vi "run_pharmaBotExp_v1.000.vi"(0 "data in":T12={"daq_ao 1"="Dev1/ao0", "daq_ai 1"="Dev1/ai0", "experiment day folder"=path "C:/multiBot/data/debug/testing", "Multiclamp init error"=0, "Multiclamp Handle Out"=10225184, "sampling rate (Hz)"=20000, "trial name"="t1"}, 1 "auto run?":bool, 3 "which manipulator":T13(ring), 4 "HEK/slice options":enum16{"slice", "HEK"}(ring), 5 "error in":errorcluster, 6 "Validate after Experiment":bool, 7 "common cluster":T9, 11 "individual controls in":T8, 13 "images":T3={"slice image"="remote image 00000000137F745C", "pipette template"="remote image 00000000137F7D5C", "found pipette"=refnum, "pipette mask for cell tracker"=refnum, "cell images ref"=refnum}) -> (10 "Cell Looks Good?":bool=TRUE, 12 "ValidationOutputCluster":T5(array[cluster]), 14 "ValidationResults":waveform(dbl)[][](array[waveform]), 15 "ValidationPos1":T6(array[ring]), 16 "Exp. Terminated":bool, 17 "ValidationPos2":T6(array[ring]), 18 "ValidationWaveform":waveform(dbl)[](array[waveform]), 19 "error out":errorcluster)   [LabVIEW 2019] (continued)
                  }
                  frame True {
                    n489 = local write "Current Position"(w583) -> ()
                  }
                }
              }
              frame #3 {
                n490 = Unbundle By Name(w601) -> ("JumperPositions.JumperPos A"=w600:refnum<vi>)
                n491 = property class="Arr (strict)"(reference=w600) -> ("Value"=w584:dbl[], "Caption.Text"=w589:string)  [unwired: 1 in, 2 out]
                n492 = Index Array(array=w587) -> (element #1=w598:i32, element #2=w596:i32, element #3=w595:i32)  [unwired: 3 in]
                n493 = Divide(x=w584, y=10) -> (x/y=w585:dbl[])
                n494 = To Long Integer(number=w585) -> (32bit integer=w586:i32[])
                n495 = Index Array(array=w586) -> (element #1=w599:i32, element #2=w597:i32, element #3=w594:i32)  [unwired: 3 in]
                n496 = Equal?(x=w599, y=w598) -> (x = y?=w593:bool)
                n497 = Equal?(x=w597, y=w596) -> (x = y?=w592:bool)
                n498 = Equal?(x=w594, y=w595) -> (x = y?=w591:bool)
                n499 = Compound Arithmetic op=AND(w593, w592, w591) -> (w590:bool)
                n500 = case shown="True" w590 {
                  tunnel: w589 -> [_ w602]
                  frame False {
                  }
                  frame True {
                    n501 = local write "Current Position"(w602) -> ()
                  }
                }
              }
              frame #4 {
                n502 = Unbundle By Name(w620) -> ("JumperPositions.JumperPos B"=w619:refnum<vi>)
                n503 = property class="Arr (strict)"(reference=w619) -> ("Value"=w605:dbl[], "Caption.Text"=w608:string)  [unwired: 1 in, 2 out]
                n504 = Index Array(array=w603) -> (element #1=w617:i32, element #2=w615:i32, element #3=w614:i32)  [unwired: 3 in]
                n505 = Divide(x=w605, y=10) -> (x/y=w606:dbl[])
                n506 = To Long Integer(number=w606) -> (32bit integer=w604:i32[])
                n507 = Index Array(array=w604) -> (element #1=w618:i32, element #2=w616:i32, element #3=w613:i32)  [unwired: 3 in]
                n508 = Equal?(x=w618, y=w617) -> (x = y?=w612:bool)
                n509 = Equal?(x=w616, y=w615) -> (x = y?=w611:bool)
                n510 = Equal?(x=w613, y=w614) -> (x = y?=w610:bool)
                n511 = Compound Arithmetic op=AND(w612, w611, w610) -> (w609:bool)
                n512 = case shown="True" w609 {
                  tunnel: w608 -> [_ w621]
                  frame False {
                  }
                  frame True {
                    n513 = local write "Current Position"(w621) -> ()
                  }
                }
              }
              frame #5 {
                n514 = Unbundle By Name(w639) -> ("JumperPositions.JumperPos C"=w638:refnum<vi>)
                n515 = property class="Arr (strict)"(reference=w638) -> ("Value"=w624:dbl[], "Caption.Text"=w627:string)  [unwired: 1 in, 2 out]
                n516 = Index Array(array=w622) -> (element #1=w636:i32, element #2=w634:i32, element #3=w633:i32)  [unwired: 3 in]
                n517 = Divide(x=w624, y=10) -> (x/y=w625:dbl[])
                n518 = To Long Integer(number=w625) -> (32bit integer=w623:i32[])
                n519 = Index Array(array=w623) -> (element #1=w637:i32, element #2=w635:i32, element #3=w632:i32)  [unwired: 3 in]
                n520 = Equal?(x=w637, y=w636) -> (x = y?=w631:bool)
                n521 = Equal?(x=w635, y=w634) -> (x = y?=w630:bool)
                n522 = Equal?(x=w632, y=w633) -> (x = y?=w629:bool)
                n523 = Compound Arithmetic op=AND(w631, w630, w629) -> (w628:bool)
                n524 = case shown="True" w628 {
                  tunnel: w627 -> [_ w640]
                  frame False {
                  }
                  frame True {
                    n525 = local write "Current Position"(w640) -> ()
                  }
                }
              }
              frame #6 {
                n526 = Unbundle By Name(w658) -> ("JumperPositions.JumperPos o-A"=w657:refnum<vi>)
                n527 = property class="Arr (strict)"(reference=w657) -> ("Value"=w643:dbl[], "Caption.Text"=w646:string)  [unwired: 1 in, 2 out]
                n528 = Index Array(array=w641) -> (element #1=w655:i32, element #2=w653:i32, element #3=w652:i32)  [unwired: 3 in]
                n529 = Divide(x=w643, y=10) -> (x/y=w644:dbl[])
                n530 = To Long Integer(number=w644) -> (32bit integer=w642:i32[])
                n531 = Index Array(array=w642) -> (element #1=w656:i32, element #2=w654:i32, element #3=w651:i32)  [unwired: 3 in]
                n532 = Equal?(x=w656, y=w655) -> (x = y?=w650:bool)
                n533 = Equal?(x=w654, y=w653) -> (x = y?=w649:bool)
                n534 = Equal?(x=w651, y=w652) -> (x = y?=w648:bool)
                n535 = Compound Arithmetic op=AND(w650, w649, w648) -> (w647:bool)
                n536 = case shown="True" w647 {
                  tunnel: w646 -> [_ w659]
                  frame False {
                  }
                  frame True {
                    n537 = local write "Current Position"(w659) -> ()
                  }
                }
              }
              frame #7 {
                n538 = Unbundle By Name(w677) -> ("JumperPositions.JumperPos A-o"=w676:refnum<vi>)
                n539 = property class="Arr (strict)"(reference=w676) -> ("Value"=w662:dbl[], "Caption.Text"=w665:string)  [unwired: 1 in, 2 out]
                n540 = Index Array(array=w660) -> (element #1=w674:i32, element #2=w672:i32, element #3=w671:i32)  [unwired: 3 in]
                n541 = Divide(x=w662, y=10) -> (x/y=w663:dbl[])
                n542 = To Long Integer(number=w663) -> (32bit integer=w661:i32[])
                n543 = Index Array(array=w661) -> (element #1=w675:i32, element #2=w673:i32, element #3=w670:i32)  [unwired: 3 in]
                n544 = Equal?(x=w675, y=w674) -> (x = y?=w669:bool)
                n545 = Equal?(x=w673, y=w672) -> (x = y?=w668:bool)
                n546 = Equal?(x=w670, y=w671) -> (x = y?=w667:bool)
                n547 = Compound Arithmetic op=AND(w669, w668, w667) -> (w666:bool)
                n548 = case shown="True" w666 {
                  tunnel: w665 -> [_ w678]
                  frame False {
                  }
                  frame True {
                    n549 = local write "Current Position"(w678) -> ()
                  }
                }
              }
              frame #8 {
                n550 = Unbundle By Name(w696) -> ("JumperPositions.JumperPos A-B"=w695:refnum<vi>)
                n551 = property class="Arr (strict)"(reference=w695) -> ("Value"=w681:dbl[], "Caption.Text"=w684:string)  [unwired: 1 in, 2 out]
                n552 = Index Array(array=w679) -> (element #1=w693:i32, element #2=w691:i32, element #3=w690:i32)  [unwired: 3 in]
                n553 = Divide(x=w681, y=10) -> (x/y=w682:dbl[])
                n554 = To Long Integer(number=w682) -> (32bit integer=w680:i32[])
                n555 = Index Array(array=w680) -> (element #1=w694:i32, element #2=w692:i32, element #3=w689:i32)  [unwired: 3 in]
                n556 = Equal?(x=w694, y=w693) -> (x = y?=w688:bool)
                n557 = Equal?(x=w692, y=w691) -> (x = y?=w687:bool)
                n558 = Equal?(x=w689, y=w690) -> (x = y?=w686:bool)
                n559 = Compound Arithmetic op=AND(w688, w687, w686) -> (w685:bool)
                n560 = case shown="True" w685 {
                  tunnel: w684 -> [_ w697]
                  frame False {
                  }
                  frame True {
                    n561 = local write "Current Position"(w697) -> ()
                  }
                }
              }
              frame #9 {
                n562 = Unbundle By Name(w715) -> ("JumperPositions.JumperPos B-A"=w714:refnum<vi>)
                n563 = property class="Arr (strict)"(reference=w714) -> ("Value"=w700:dbl[], "Caption.Text"=w703:string)  [unwired: 1 in, 2 out]
                n564 = Index Array(array=w698) -> (element #1=w712:i32, element #2=w710:i32, element #3=w709:i32)  [unwired: 3 in]
                n565 = Divide(x=w700, y=10) -> (x/y=w701:dbl[])
                n566 = To Long Integer(number=w701) -> (32bit integer=w699:i32[])
                n567 = Index Array(array=w699) -> (element #1=w713:i32, element #2=w711:i32, element #3=w708:i32)  [unwired: 3 in]
                n568 = Equal?(x=w713, y=w712) -> (x = y?=w707:bool)
                n569 = Equal?(x=w711, y=w710) -> (x = y?=w706:bool)
                n570 = Equal?(x=w708, y=w709) -> (x = y?=w705:bool)
                n571 = Compound Arithmetic op=AND(w707, w706, w705) -> (w704:bool)
                n572 = case shown="True" w704 {
                  tunnel: w703 -> [_ w716]
                  frame False {
                  }
                  frame True {
                    n573 = local write "Current Position"(w716) -> ()
                  }
                }
              }
              frame #10 {
                n574 = Unbundle By Name(w734) -> ("JumperPositions.JumperPos B-C"=w733:refnum<vi>)
                n575 = property class="Arr (strict)"(reference=w733) -> ("Value"=w719:dbl[], "Caption.Text"=w722:string)  [unwired: 1 in, 2 out]
                n576 = Index Array(array=w717) -> (element #1=w731:i32, element #2=w729:i32, element #3=w728:i32)  [unwired: 3 in]
                n577 = Divide(x=w719, y=10) -> (x/y=w720:dbl[])
                n578 = To Long Integer(number=w720) -> (32bit integer=w718:i32[])
                n579 = Index Array(array=w718) -> (element #1=w732:i32, element #2=w730:i32, element #3=w727:i32)  [unwired: 3 in]
                n580 = Equal?(x=w732, y=w731) -> (x = y?=w726:bool)
                n581 = Equal?(x=w730, y=w729) -> (x = y?=w725:bool)
                n582 = Equal?(x=w727, y=w728) -> (x = y?=w724:bool)
                n583 = Compound Arithmetic op=AND(w726, w725, w724) -> (w723:bool)
                n584 = case shown="True" w723 {
                  tunnel: w722 -> [_ w735]
                  frame False {
                  }
                  frame True {
                    n585 = local write "Current Position"(w735) -> ()
                  }
                }
              }
              frame #11 {
                n586 = Unbundle By Name(w753) -> ("JumperPositions.JumperPos C-B"=w752:refnum<vi>)
                n587 = property class="Arr (strict)"(reference=w752) -> ("Value"=w738:dbl[], "Caption.Text"=w741:string)  [unwired: 1 in, 2 out]
                n588 = Index Array(array=w736) -> (element #1=w750:i32, element #2=w748:i32, element #3=w747:i32)  [unwired: 3 in]
                n589 = Divide(x=w738, y=10) -> (x/y=w739:dbl[])
                n590 = To Long Integer(number=w739) -> (32bit integer=w737:i32[])
                n591 = Index Array(array=w737) -> (element #1=w751:i32, element #2=w749:i32, element #3=w746:i32)  [unwired: 3 in]
                n592 = Equal?(x=w751, y=w750) -> (x = y?=w745:bool)
                n593 = Equal?(x=w749, y=w748) -> (x = y?=w744:bool)
                n594 = Equal?(x=w746, y=w747) -> (x = y?=w743:bool)
                n595 = Compound Arithmetic op=AND(w745, w744, w743) -> (w742:bool)
                n596 = case shown="True" w742 {
                  tunnel: w741 -> [_ w754]
                  frame False {
                  }
                  frame True {
                    n597 = local write "Current Position"(w754) -> ()
                  }
                }
              }
              frame #12 {
                n598 = Unbundle By Name(w772) -> ("JumperPositions.JumperPos C-o"=w771:refnum<vi>)
                n599 = property class="Arr (strict)"(reference=w771) -> ("Value"=w757:dbl[], "Caption.Text"=w760:string)  [unwired: 1 in, 2 out]
                n600 = Index Array(array=w755) -> (element #1=w769:i32, element #2=w767:i32, element #3=w766:i32)  [unwired: 3 in]
                n601 = Divide(x=w757, y=10) -> (x/y=w758:dbl[])
                n602 = To Long Integer(number=w758) -> (32bit integer=w756:i32[])
                n603 = Index Array(array=w756) -> (element #1=w770:i32, element #2=w768:i32, element #3=w765:i32)  [unwired: 3 in]
                n604 = Equal?(x=w770, y=w769) -> (x = y?=w764:bool)
                n605 = Equal?(x=w768, y=w767) -> (x = y?=w763:bool)
                n606 = Equal?(x=w765, y=w766) -> (x = y?=w762:bool)
                n607 = Compound Arithmetic op=AND(w764, w763, w762) -> (w761:bool)
                n608 = case shown="True" w761 {
                  tunnel: w760 -> [_ w773]
                  frame False {
                  }
                  frame True {
                    n609 = local write "Current Position"(w773) -> ()
                  }
                }
              }
              frame #13 {
                n610 = Unbundle By Name(w791) -> ("JumperPositions.JumperPos o-C"=w790:refnum<vi>)
                n611 = property class="Arr (strict)"(reference=w790) -> ("Value"=w776:dbl[], "Caption.Text"=w779:string)  [unwired: 1 in, 2 out]
                n612 = Index Array(array=w774) -> (element #1=w788:i32, element #2=w786:i32, element #3=w785:i32)  [unwired: 3 in]
                n613 = Divide(x=w776, y=10) -> (x/y=w777:dbl[])
                n614 = To Long Integer(number=w777) -> (32bit integer=w775:i32[])
                n615 = Index Array(array=w775) -> (element #1=w789:i32, element #2=w787:i32, element #3=w784:i32)  [unwired: 3 in]
                n616 = Equal?(x=w789, y=w788) -> (x = y?=w783:bool)
                n617 = Equal?(x=w787, y=w786) -> (x = y?=w782:bool)
                n618 = Equal?(x=w784, y=w785) -> (x = y?=w781:bool)
                n619 = Compound Arithmetic op=AND(w783, w782, w781) -> (w780:bool)
                n620 = case shown="True" w780 {
                  tunnel: w779 -> [_ w792]
                  frame False {
                  }
                  frame True {
                    n621 = local write "Current Position"(w792) -> ()
                  }
                }
              }
            }
          }
        }
        n622 = local read "Running"() -> (w526:bool)
        n623 = local read "Experiment Done"() -> (w522:bool)
        n624 = Not(x=w526) -> (.not. x?=w525:bool)
        n625 = Or(x=w522, y=w525) -> (x .or. y?=w523:bool)
        n626 = Wait (ms)(milliseconds to wait=u32 100) -> ()  [unwired: 1 out]
      }
      frame True {
        n627 = Wait (ms)(milliseconds to wait=u32 10000) -> ()  [unwired: 1 out]
      }
    }
  }
  n628 = control-ref of="PhaseK Experiment Option"() -> (w360:refnum<vi>)
  n629 = control-ref of="PhaseE Experiment Option"() -> (w436:refnum<vi>)
  n630 = control-ref of="Paired Pulse E"() -> (w242:refnum<vi>)
  n631 = control-ref of="Jump Train E"() -> (w241:refnum<vi>)
  n632 = control-ref of="Voltage Ramp E"() -> (w240:refnum<vi>)
  n633 = control-ref of="Voltage Step E"() -> (w239:refnum<vi>)
  n634 = control-ref of="Solution Change E"() -> (w238:refnum<vi>)
  n635 = control-ref of="Single Jump E"() -> (w237:refnum<vi>)
  n636 = control-ref of="Single Manip Jump E"() -> (w236:refnum<vi>)
  n637 = control-ref of="Gap Free E"() -> (w235:refnum<vi>)
  n638 = control-ref of="Multi Manip Jump E"() -> (w234:refnum<vi>)
  n639 = control-ref of="Voltage Pulse E"() -> (w233:refnum<vi>)
  n640 = control-ref of="Current Pulse E"() -> (w52:refnum<vi>)
  n641 = control-ref of="Current Ramp E"() -> (w51:refnum<vi>)
  n642 = control-ref of="Gap Free Iclamp E"() -> (w50:refnum<vi>)
  n643 = Bundle(cluster=T34 {"Phase A Done"=refnum, "Phase B Done"=refnum, "Phase C Done"=refnum, "Phase D Done"=refnum, "Phase E Done"=refnum, "Phase F Done"=refnum, "Phase G Done"=refnum, "Phase H Done"=refnum, "Phase I Done"=refnum, "Phase J Done"=refnum, "Phase K Done"=refnum, "Phase L Done"=refnum} ("PhaseStatusCluster"), "Phase A Done"=w337, "Phase B Done"=w336, "Phase C Done"=w335, "Phase D Done"=w334, "Phase E Done"=w333, "Phase F Done"=w332, "Phase G Done"=w331, "Phase H Done"=w330, "Phase I Done"=w329, "Phase J Done"=w328, "Phase K Done"=w327, "Phase L Done"=w326) -> (w324:T34)
  n644 = Bundle(cluster="PhaseX Cluster", "Phase Experiment Option"=w360, "Paired Pulse"=w172, "Jump Train"=w171, "Voltage Ramp"=w170, "Voltage Step"=w169, "Solution Change"=w168, "Single Jump"=w167, "Single Manip Jump"=w166, "Gap Free"=w165, "Multi Manip Jump"=w164, "Voltage Pulse"=w163, "Current Pulse"=w46, "Current Ramp"=w45, "Gap Free Iclamp"=w44) -> (w354:T1)
  n645 = Bundle(cluster="PhaseX Cluster", "Phase Experiment Option"=w436, "Paired Pulse"=w242, "Jump Train"=w241, "Voltage Ramp"=w240, "Voltage Step"=w239, "Solution Change"=w238, "Single Jump"=w237, "Single Manip Jump"=w236, "Gap Free"=w235, "Multi Manip Jump"=w234, "Voltage Pulse"=w233, "Current Pulse"=w52, "Current Ramp"=w51, "Gap Free Iclamp"=w50) -> (w433:T1)
  n646 = control-ref of="Paired Pulse L"() -> (w162:refnum<vi>)
  n647 = control-ref of="Single Manip Jump L"() -> (w156:refnum<vi>)
  n648 = control-ref of="Voltage Ramp L"() -> (w160:refnum<vi>)
  n649 = control-ref of="Voltage Step L"() -> (w159:refnum<vi>)
  n650 = control-ref of="Solution Change L"() -> (w158:refnum<vi>)
  n651 = control-ref of="Single Jump L"() -> (w157:refnum<vi>)
  n652 = control-ref of="Jump Train L"() -> (w161:refnum<vi>)
  n653 = control-ref of="Gap Free L"() -> (w155:refnum<vi>)
  n654 = control-ref of="Multi Manip Jump L"() -> (w154:refnum<vi>)
  n655 = control-ref of="Voltage Pulse L"() -> (w153:refnum<vi>)
  n656 = control-ref of="Current Pulse L"() -> (w43:refnum<vi>)
  n657 = control-ref of="Current Ramp L"() -> (w42:refnum<vi>)
  n658 = control-ref of="Gap Free Iclamp L"() -> (w41:refnum<vi>)
  n659 = control-ref of="PhaseL Experiment Option"() -> (w359:refnum<vi>)
  n660 = control-ref of="Current Pulse F"() -> (w49:refnum<vi>)
  n661 = control-ref of="Current Ramp F"() -> (w48:refnum<vi>)
  n662 = control-ref of="Gap Free Iclamp F"() -> (w47:refnum<vi>)
  n663 = control-ref of="Paired Pulse F"() -> (w222:refnum<vi>)
  n664 = control-ref of="Jump Train F"() -> (w221:refnum<vi>)
  n665 = control-ref of="Voltage Ramp F"() -> (w220:refnum<vi>)
  n666 = control-ref of="Voltage Step F"() -> (w219:refnum<vi>)
  n667 = control-ref of="Solution Change F"() -> (w218:refnum<vi>)
  n668 = control-ref of="Single Jump F"() -> (w217:refnum<vi>)
  n669 = control-ref of="Single Manip Jump F"() -> (w216:refnum<vi>)
  n670 = control-ref of="Gap Free F"() -> (w215:refnum<vi>)
  n671 = control-ref of="Multi Manip Jump F"() -> (w214:refnum<vi>)
  n672 = control-ref of="Voltage Pulse F"() -> (w213:refnum<vi>)
  n673 = control-ref of="PhaseF Experiment Option"() -> (w435:refnum<vi>)
  n674 = Bundle(cluster="PhaseX Cluster", "Phase Experiment Option"=w359, "Paired Pulse"=w162, "Jump Train"=w161, "Voltage Ramp"=w160, "Voltage Step"=w159, "Solution Change"=w158, "Single Jump"=w157, "Single Manip Jump"=w156, "Gap Free"=w155, "Multi Manip Jump"=w154, "Voltage Pulse"=w153, "Current Pulse"=w43, "Current Ramp"=w42, "Gap Free Iclamp"=w41) -> (w353:T1)
  n675 = Bundle(cluster="PhaseX Cluster", "Phase Experiment Option"=w435, "Paired Pulse"=w222, "Jump Train"=w221, "Voltage Ramp"=w220, "Voltage Step"=w219, "Solution Change"=w218, "Single Jump"=w217, "Single Manip Jump"=w216, "Gap Free"=w215, "Multi Manip Jump"=w214, "Voltage Pulse"=w213, "Current Pulse"=w49, "Current Ramp"=w48, "Gap Free Iclamp"=w47) -> (w432:T1)
  n676 = Bundle(cluster="ExperimentOptionsCluster", "How Many Experimental Phases?"=w451, "PhaseA Cluster"=w450, "PhaseB Cluster"=w449, "PhaseC Cluster"=w445, "PhaseD Cluster"=w434, "PhaseE Cluster"=w433, "PhaseF Cluster"=w432, "time to wait for solution change (min)"=w428, "valve Time Cluster"=w423, "PhaseG Cluster"=w358, "PhaseH Cluster"=w357, "PhaseI Cluster"=w356, "PhaseJ Cluster"=w355, "PhaseK Cluster"=w354, "PhaseL Cluster"=w353, "PhaseStatusCluster"=w324) -> (w78:T2)
  n677 = while {
    tunnel: w481 -> [w801]
    tunnel: w480 -> [w800]
    tunnel: w474 -> [w813]
    tunnel: w476 -> [w812]
    tunnel: "common cluster" -> [w806]
    tunnel: "individual controls in" -> [w810]
    tunnel: "images" -> [w809]
    tunnel: "which manipulator" -> [w808]
    tunnel: w78 -> [w807]
    tunnel: w441 -> [w802]
    tunnel: w378 -> [w799]
    tunnel: w377 -> [w798]
    stop <- w805 stop-if-true
    # "Experiment"
    # "images"
    # "individual"
    # "Common"
    n678 = case shown="True" "auto WC run trigger" {
      selector: "auto WC run trigger" -> [_ w841]
      tunnel: w813 -> [_ w845]
      tunnel: w812 -> [_ w869]
      tunnel: [w819 w835] -> w796
      tunnel: errorcluster {"status"=FALSE, "code"=0, "source"=""} ("error in") -> [w819 w838]
      tunnel: w806 -> [_ w833]
      tunnel: w810 -> [_ w895]
      tunnel: w809 -> [_ w896]
      tunnel: w808 -> [_ w894]
      tunnel: w807 -> [_ w824]
      tunnel: [FALSE ("Experiment Done") w888] -> w804
      tunnel: w802 -> [_ w885]
      tunnel: w801 -> [_ w880]
      tunnel: w800 -> [_ w879]
      tunnel: w799 -> [_ w858]
      tunnel: w798 -> [_ w854]
      frame False {
        # "if not running auto WC, wait 200 ms"
        n679 = local read "Puase for Loading"() -> (w816:bool)
        n680 = Select(t=u32 10000, s=w816, f=u32 200 ("milliseconds to wait")) -> (s? t:f=w817:u32)
        n681 = Wait (ms)(milliseconds to wait=w817) -> ()  [unwired: 1 out]
      }
      frame True {
        # "write the whole config to the experiment day folder"
        n682 = local read "How Many Experimental Phases?"() -> (w840:i32)
        n683 = local write "Exp Started"(w841) -> ()
        n684 = case shown="1" w840 {
          tunnel: [w931 w932 w947 w963 w980 w998 w1017 w1037 w1058 w1080 w1103 w1127 w1152] -> w839
          tunnel: w838 -> [w931 w932 w947 w963 w980 w998 w1017 w1037 w1058 w1080 w1103 w1127 w1152]
          frame 0, Default {
          }
          frame 1 {
            w933 = "" ("Phase F Exp Option")
            n685 = local read "PhaseA Experiment Option"() -> (w945:string)
            n686 = local write "Phase A Exp Option"(w945) -> ()
            n687 = local write "Phase B Exp Option"(w933) -> ()
            n688 = local write "Phase D Exp Option"(w933) -> ()
            n689 = local write "Phase C Exp Option"(w933) -> ()
            n690 = local write "Phase E Exp Option"(w933) -> ()
            n691 = local write "Phase F Exp Option"(w933) -> ()
            n692 = local write "Phase A"(TRUE ("Phase A")) -> ()
            n693 = local write "Phase C"(FALSE ("Phase A")) -> ()
            n694 = local write "Phase D"(FALSE ("Phase A")) -> ()
            n695 = local write "Phase B"(FALSE ("Phase A")) -> ()
            n696 = local write "Phase E"(FALSE ("Phase A")) -> ()
            n697 = local write "Phase F"(FALSE ("Phase A")) -> ()
            n698 = local write "Phase L Exp Option"(w933) -> ()
            n699 = local write "Phase K Exp Option"(w933) -> ()
            n700 = local write "Phase J Exp Option"(w933) -> ()
            n701 = local write "Phase I Exp Option"(w933) -> ()
            n702 = local write "Phase H Exp Option"(w933) -> ()
            n703 = local write "Phase G Exp Option"(w933) -> ()
            n704 = local write "Phase L"(FALSE ("Phase A")) -> ()
            n705 = local write "Phase K"(FALSE ("Phase A")) -> ()
            n706 = local write "Phase J"(FALSE ("Phase A")) -> ()
            n707 = local write "Phase I"(FALSE ("Phase A")) -> ()
            n708 = local write "Phase H"(FALSE ("Phase A")) -> ()
            n709 = local write "Phase G"(FALSE ("Phase A")) -> ()
          }
          frame 2 {
            w949 = "" ("Phase F Exp Option")
            n710 = local read "PhaseA Experiment Option"() -> (w961:string)
            n711 = local read "PhaseB Experiment Option"() -> (w948:string)
            n712 = local write "Phase A Exp Option"(w961) -> ()
            n713 = local write "Phase B Exp Option"(w948) -> ()
            n714 = local write "Phase D Exp Option"(w949) -> ()
            n715 = local write "Phase C Exp Option"(w949) -> ()
            n716 = local write "Phase E Exp Option"(w949) -> ()
            n717 = local write "Phase F Exp Option"(w949) -> ()
            n718 = local write "Phase A"(TRUE ("Phase A")) -> ()
            n719 = local write "Phase C"(FALSE ("Phase A")) -> ()
            n720 = local write "Phase D"(FALSE ("Phase A")) -> ()
            n721 = local write "Phase B"(TRUE ("Phase A")) -> ()
            n722 = local write "Phase E"(FALSE ("Phase A")) -> ()
            n723 = local write "Phase F"(FALSE ("Phase A")) -> ()
            n724 = local write "Phase L Exp Option"(w949) -> ()
            n725 = local write "Phase K Exp Option"(w949) -> ()
            n726 = local write "Phase J Exp Option"(w949) -> ()
            n727 = local write "Phase I Exp Option"(w949) -> ()
            n728 = local write "Phase H Exp Option"(w949) -> ()
            n729 = local write "Phase G Exp Option"(w949) -> ()
            n730 = local write "Phase L"(FALSE ("Phase A")) -> ()
            n731 = local write "Phase K"(FALSE ("Phase A")) -> ()
            n732 = local write "Phase J"(FALSE ("Phase A")) -> ()
            n733 = local write "Phase I"(FALSE ("Phase A")) -> ()
            n734 = local write "Phase H"(FALSE ("Phase A")) -> ()
            n735 = local write "Phase G"(FALSE ("Phase A")) -> ()
          }
          frame 3 {
            w966 = "" ("Phase F Exp Option")
            n736 = local read "PhaseA Experiment Option"() -> (w978:string)
            n737 = local read "PhaseB Experiment Option"() -> (w965:string)
            n738 = local read "PhaseC Experiment Option"() -> (w964:string)
            n739 = local write "Phase A Exp Option"(w978) -> ()
            n740 = local write "Phase B Exp Option"(w965) -> ()
            n741 = local write "Phase D Exp Option"(w966) -> ()
            n742 = local write "Phase C Exp Option"(w964) -> ()
            n743 = local write "Phase E Exp Option"(w966) -> ()
            n744 = local write "Phase F Exp Option"(w966) -> ()
            n745 = local write "Phase A"(TRUE ("Phase A")) -> ()
            n746 = local write "Phase C"(TRUE ("Phase A")) -> ()
            n747 = local write "Phase D"(FALSE ("Phase A")) -> ()
            n748 = local write "Phase B"(TRUE ("Phase A")) -> ()
            n749 = local write "Phase E"(FALSE ("Phase A")) -> ()
            n750 = local write "Phase F"(FALSE ("Phase A")) -> ()
            n751 = local write "Phase L Exp Option"(w966) -> ()
            n752 = local write "Phase K Exp Option"(w966) -> ()
            n753 = local write "Phase J Exp Option"(w966) -> ()
            n754 = local write "Phase I Exp Option"(w966) -> ()
            n755 = local write "Phase H Exp Option"(w966) -> ()
            n756 = local write "Phase G Exp Option"(w966) -> ()
            n757 = local write "Phase L"(FALSE ("Phase A")) -> ()
            n758 = local write "Phase K"(FALSE ("Phase A")) -> ()
            n759 = local write "Phase J"(FALSE ("Phase A")) -> ()
            n760 = local write "Phase I"(FALSE ("Phase A")) -> ()
            n761 = local write "Phase H"(FALSE ("Phase A")) -> ()
            n762 = local write "Phase G"(FALSE ("Phase A")) -> ()
          }
          frame 4 {
            w984 = "" ("Phase F Exp Option")
            n763 = local read "PhaseA Experiment Option"() -> (w996:string)
            n764 = local read "PhaseB Experiment Option"() -> (w983:string)
            n765 = local read "PhaseC Experiment Option"() -> (w982:string)
            n766 = local read "PhaseD Experiment Option"() -> (w981:string)
            n767 = local write "Phase A Exp Option"(w996) -> ()
            n768 = local write "Phase B Exp Option"(w983) -> ()
            n769 = local write "Phase D Exp Option"(w981) -> ()
            n770 = local write "Phase C Exp Option"(w982) -> ()
            n771 = local write "Phase E Exp Option"(w984) -> ()
            n772 = local write "Phase F Exp Option"(w984) -> ()
            n773 = local write "Phase A"(TRUE ("Phase A")) -> ()
            n774 = local write "Phase C"(TRUE ("Phase A")) -> ()
            n775 = local write "Phase D"(TRUE ("Phase A")) -> ()
            n776 = local write "Phase B"(TRUE ("Phase A")) -> ()
            n777 = local write "Phase E"(FALSE ("Phase A")) -> ()
            n778 = local write "Phase F"(FALSE ("Phase A")) -> ()
            n779 = local write "Phase L Exp Option"(w984) -> ()
            n780 = local write "Phase K Exp Option"(w984) -> ()
            n781 = local write "Phase J Exp Option"(w984) -> ()
            n782 = local write "Phase I Exp Option"(w984) -> ()
            n783 = local write "Phase H Exp Option"(w984) -> ()
            n784 = local write "Phase G Exp Option"(w984) -> ()
            n785 = local write "Phase L"(FALSE ("Phase A")) -> ()
            n786 = local write "Phase K"(FALSE ("Phase A")) -> ()
            n787 = local write "Phase J"(FALSE ("Phase A")) -> ()
            n788 = local write "Phase I"(FALSE ("Phase A")) -> ()
            n789 = local write "Phase H"(FALSE ("Phase A")) -> ()
            n790 = local write "Phase G"(FALSE ("Phase A")) -> ()
          }
          frame 5 {
            w1003 = "" ("Phase F Exp Option")
            n791 = local read "PhaseA Experiment Option"() -> (w1015:string)
            n792 = local read "PhaseB Experiment Option"() -> (w1002:string)
            n793 = local read "PhaseC Experiment Option"() -> (w1001:string)
            n794 = local read "PhaseD Experiment Option"() -> (w1000:string)
            n795 = local read "PhaseE Experiment Option"() -> (w999:string)
            n796 = local write "Phase A Exp Option"(w1015) -> ()
            n797 = local write "Phase B Exp Option"(w1002) -> ()
            n798 = local write "Phase D Exp Option"(w1000) -> ()
            n799 = local write "Phase C Exp Option"(w1001) -> ()
            n800 = local write "Phase E Exp Option"(w999) -> ()
            n801 = local write "Phase F Exp Option"(w1003) -> ()
            n802 = local write "Phase A"(TRUE ("Phase A")) -> ()
            n803 = local write "Phase C"(TRUE ("Phase A")) -> ()
            n804 = local write "Phase D"(TRUE ("Phase A")) -> ()
            n805 = local write "Phase B"(TRUE ("Phase A")) -> ()
            n806 = local write "Phase E"(TRUE ("Phase A")) -> ()
            n807 = local write "Phase F"(FALSE ("Phase A")) -> ()
            n808 = local write "Phase L Exp Option"(w1003) -> ()
            n809 = local write "Phase K Exp Option"(w1003) -> ()
            n810 = local write "Phase J Exp Option"(w1003) -> ()
            n811 = local write "Phase I Exp Option"(w1003) -> ()
            n812 = local write "Phase H Exp Option"(w1003) -> ()
            n813 = local write "Phase G Exp Option"(w1003) -> ()
            n814 = local write "Phase L"(FALSE ("Phase A")) -> ()
            n815 = local write "Phase K"(FALSE ("Phase A")) -> ()
            n816 = local write "Phase J"(FALSE ("Phase A")) -> ()
            n817 = local write "Phase I"(FALSE ("Phase A")) -> ()
            n818 = local write "Phase H"(FALSE ("Phase A")) -> ()
            n819 = local write "Phase G"(FALSE ("Phase A")) -> ()
          }
          frame 6 {
            w1023 = "" ("Phase F Exp Option")
            n820 = local read "PhaseA Experiment Option"() -> (w1035:string)
            n821 = local read "PhaseB Experiment Option"() -> (w1022:string)
            n822 = local read "PhaseC Experiment Option"() -> (w1021:string)
            n823 = local read "PhaseD Experiment Option"() -> (w1020:string)
            n824 = local read "PhaseE Experiment Option"() -> (w1019:string)
            n825 = local read "PhaseF Experiment Option"() -> (w1018:string)
            n826 = local write "Phase A Exp Option"(w1035) -> ()
            n827 = local write "Phase B Exp Option"(w1022) -> ()
            n828 = local write "Phase D Exp Option"(w1020) -> ()
            n829 = local write "Phase C Exp Option"(w1021) -> ()
            n830 = local write "Phase E Exp Option"(w1019) -> ()
            n831 = local write "Phase F Exp Option"(w1018) -> ()
            n832 = local write "Phase A"(TRUE ("Phase A")) -> ()
            n833 = local write "Phase C"(TRUE ("Phase A")) -> ()
            n834 = local write "Phase D"(TRUE ("Phase A")) -> ()
            n835 = local write "Phase B"(TRUE ("Phase A")) -> ()
            n836 = local write "Phase E"(TRUE ("Phase A")) -> ()
            n837 = local write "Phase F"(TRUE ("Phase A")) -> ()
            n838 = local write "Phase L Exp Option"(w1023) -> ()
            n839 = local write "Phase K Exp Option"(w1023) -> ()
            n840 = local write "Phase J Exp Option"(w1023) -> ()
            n841 = local write "Phase I Exp Option"(w1023) -> ()
            n842 = local write "Phase H Exp Option"(w1023) -> ()
            n843 = local write "Phase G Exp Option"(w1023) -> ()
            n844 = local write "Phase L"(FALSE ("Phase A")) -> ()
            n845 = local write "Phase K"(FALSE ("Phase A")) -> ()
            n846 = local write "Phase J"(FALSE ("Phase A")) -> ()
            n847 = local write "Phase I"(FALSE ("Phase A")) -> ()
            n848 = local write "Phase H"(FALSE ("Phase A")) -> ()
            n849 = local write "Phase G"(FALSE ("Phase A")) -> ()
          }
          frame 7 {
            w1044 = "" ("Phase F Exp Option")
            n850 = local read "PhaseA Experiment Option"() -> (w1056:string)
            n851 = local read "PhaseB Experiment Option"() -> (w1043:string)
            n852 = local read "PhaseC Experiment Option"() -> (w1042:string)
            n853 = local read "PhaseD Experiment Option"() -> (w1041:string)
            n854 = local read "PhaseE Experiment Option"() -> (w1040:string)
            n855 = local read "PhaseF Experiment Option"() -> (w1039:string)
            n856 = local write "Phase A Exp Option"(w1056) -> ()
            n857 = local write "Phase B Exp Option"(w1043) -> ()
            n858 = local write "Phase D Exp Option"(w1041) -> ()
            n859 = local write "Phase C Exp Option"(w1042) -> ()
            n860 = local write "Phase E Exp Option"(w1040) -> ()
            n861 = local write "Phase F Exp Option"(w1039) -> ()
            n862 = local write "Phase A"(TRUE ("Phase A")) -> ()
            n863 = local write "Phase C"(TRUE ("Phase A")) -> ()
            n864 = local write "Phase D"(TRUE ("Phase A")) -> ()
            n865 = local write "Phase B"(TRUE ("Phase A")) -> ()
            n866 = local write "Phase E"(TRUE ("Phase A")) -> ()
            n867 = local write "Phase F"(TRUE ("Phase A")) -> ()
            n868 = local read "PhaseG Experiment Option"() -> (w1038:string)
            n869 = local write "Phase L Exp Option"(w1044) -> ()
            n870 = local write "Phase K Exp Option"(w1044) -> ()
            n871 = local write "Phase J Exp Option"(w1044) -> ()
            n872 = local write "Phase I Exp Option"(w1044) -> ()
            n873 = local write "Phase G Exp Option"(w1038) -> ()
            n874 = local write "Phase H Exp Option"(w1044) -> ()
            n875 = local write "Phase L"(FALSE ("Phase A")) -> ()
            n876 = local write "Phase K"(FALSE ("Phase A")) -> ()
            n877 = local write "Phase J"(FALSE ("Phase A")) -> ()
            n878 = local write "Phase I"(FALSE ("Phase A")) -> ()
            n879 = local write "Phase H"(FALSE ("Phase A")) -> ()
            n880 = local write "Phase G"(TRUE ("Phase A")) -> ()
          }
          frame 8 {
            w1066 = "" ("Phase F Exp Option")
            n881 = local read "PhaseA Experiment Option"() -> (w1078:string)
            n882 = local read "PhaseB Experiment Option"() -> (w1065:string)
            n883 = local read "PhaseC Experiment Option"() -> (w1064:string)
            n884 = local read "PhaseD Experiment Option"() -> (w1063:string)
            n885 = local read "PhaseE Experiment Option"() -> (w1062:string)
            n886 = local read "PhaseF Experiment Option"() -> (w1061:string)
            n887 = local write "Phase A Exp Option"(w1078) -> ()
            n888 = local write "Phase B Exp Option"(w1065) -> ()
            n889 = local write "Phase D Exp Option"(w1063) -> ()
            n890 = local write "Phase C Exp Option"(w1064) -> ()
            n891 = local write "Phase E Exp Option"(w1062) -> ()
            n892 = local write "Phase F Exp Option"(w1061) -> ()
            n893 = local write "Phase A"(TRUE ("Phase A")) -> ()
            n894 = local write "Phase C"(TRUE ("Phase A")) -> ()
            n895 = local write "Phase D"(TRUE ("Phase A")) -> ()
            n896 = local write "Phase B"(TRUE ("Phase A")) -> ()
            n897 = local write "Phase E"(TRUE ("Phase A")) -> ()
            n898 = local write "Phase F"(TRUE ("Phase A")) -> ()
            n899 = local read "PhaseG Experiment Option"() -> (w1060:string)
            n900 = local write "Phase L Exp Option"(w1066) -> ()
            n901 = local read "PhaseH Experiment Option"() -> (w1059:string)
            n902 = local write "Phase K Exp Option"(w1066) -> ()
            n903 = local write "Phase J Exp Option"(w1066) -> ()
            n904 = local write "Phase I Exp Option"(w1066) -> ()
            n905 = local write "Phase G Exp Option"(w1060) -> ()
            n906 = local write "Phase H Exp Option"(w1059) -> ()
            n907 = local write "Phase L"(FALSE ("Phase A")) -> ()
            n908 = local write "Phase K"(FALSE ("Phase A")) -> ()
            n909 = local write "Phase J"(FALSE ("Phase A")) -> ()
            n910 = local write "Phase I"(FALSE ("Phase A")) -> ()
            n911 = local write "Phase H"(TRUE ("Phase A")) -> ()
            n912 = local write "Phase G"(TRUE ("Phase A")) -> ()
          }
          frame 9 {
            w1089 = "" ("Phase F Exp Option")
            n913 = local read "PhaseA Experiment Option"() -> (w1101:string)
            n914 = local read "PhaseB Experiment Option"() -> (w1088:string)
            n915 = local read "PhaseC Experiment Option"() -> (w1087:string)
            n916 = local read "PhaseD Experiment Option"() -> (w1086:string)
            n917 = local read "PhaseE Experiment Option"() -> (w1085:string)
            n918 = local read "PhaseF Experiment Option"() -> (w1084:string)
            n919 = local write "Phase A Exp Option"(w1101) -> ()
            n920 = local write "Phase B Exp Option"(w1088) -> ()
            n921 = local write "Phase D Exp Option"(w1086) -> ()
            n922 = local write "Phase C Exp Option"(w1087) -> ()
            n923 = local write "Phase E Exp Option"(w1085) -> ()
            n924 = local write "Phase F Exp Option"(w1084) -> ()
            n925 = local write "Phase A"(TRUE ("Phase A")) -> ()
            n926 = local write "Phase C"(TRUE ("Phase A")) -> ()
            n927 = local write "Phase D"(TRUE ("Phase A")) -> ()
            n928 = local write "Phase B"(TRUE ("Phase A")) -> ()
            n929 = local write "Phase E"(TRUE ("Phase A")) -> ()
            n930 = local write "Phase F"(TRUE ("Phase A")) -> ()
            n931 = local read "PhaseG Experiment Option"() -> (w1083:string)
            n932 = local write "Phase L Exp Option"(w1089) -> ()
            n933 = local read "PhaseH Experiment Option"() -> (w1082:string)
            n934 = local read "PhaseI Experiment Option"() -> (w1081:string)
            n935 = local write "Phase K Exp Option"(w1089) -> ()
            n936 = local write "Phase J Exp Option"(w1089) -> ()
            n937 = local write "Phase I Exp Option"(w1081) -> ()
            n938 = local write "Phase G Exp Option"(w1083) -> ()
            n939 = local write "Phase H Exp Option"(w1082) -> ()
            n940 = local write "Phase L"(FALSE ("Phase A")) -> ()
            n941 = local write "Phase K"(FALSE ("Phase A")) -> ()
            n942 = local write "Phase J"(FALSE ("Phase A")) -> ()
            n943 = local write "Phase I"(TRUE ("Phase A")) -> ()
            n944 = local write "Phase H"(TRUE ("Phase A")) -> ()
            n945 = local write "Phase G"(TRUE ("Phase A")) -> ()
          }
          frame 10 {
            w1113 = "" ("Phase F Exp Option")
            n946 = local read "PhaseA Experiment Option"() -> (w1125:string)
            n947 = local read "PhaseB Experiment Option"() -> (w1112:string)
            n948 = local read "PhaseC Experiment Option"() -> (w1111:string)
            n949 = local read "PhaseD Experiment Option"() -> (w1110:string)
            n950 = local read "PhaseE Experiment Option"() -> (w1109:string)
            n951 = local read "PhaseF Experiment Option"() -> (w1108:string)
            n952 = local write "Phase A Exp Option"(w1125) -> ()
            n953 = local write "Phase B Exp Option"(w1112) -> ()
            n954 = local write "Phase D Exp Option"(w1110) -> ()
            n955 = local write "Phase C Exp Option"(w1111) -> ()
            n956 = local write "Phase E Exp Option"(w1109) -> ()
            n957 = local write "Phase F Exp Option"(w1108) -> ()
            n958 = local write "Phase A"(TRUE ("Phase A")) -> ()
            n959 = local write "Phase C"(TRUE ("Phase A")) -> ()
            n960 = local write "Phase D"(TRUE ("Phase A")) -> ()
            n961 = local write "Phase B"(TRUE ("Phase A")) -> ()
            n962 = local write "Phase E"(TRUE ("Phase A")) -> ()
            n963 = local write "Phase F"(TRUE ("Phase A")) -> ()
            n964 = local read "PhaseG Experiment Option"() -> (w1107:string)
            n965 = local read "PhaseJ Experiment Option"() -> (w1104:string)
            n966 = local write "Phase L Exp Option"(w1113) -> ()
            n967 = local read "PhaseH Experiment Option"() -> (w1106:string)
            n968 = local read "PhaseI Experiment Option"() -> (w1105:string)
            n969 = local write "Phase K Exp Option"(w1113) -> ()
            n970 = local write "Phase J Exp Option"(w1104) -> ()
            n971 = local write "Phase I Exp Option"(w1105) -> ()
            n972 = local write "Phase G Exp Option"(w1107) -> ()
            n973 = local write "Phase H Exp Option"(w1106) -> ()
            n974 = local write "Phase L"(FALSE ("Phase A")) -> ()
            n975 = local write "Phase K"(FALSE ("Phase A")) -> ()
            n976 = local write "Phase J"(TRUE ("Phase A")) -> ()
            n977 = local write "Phase I"(TRUE ("Phase A")) -> ()
            n978 = local write "Phase H"(TRUE ("Phase A")) -> ()
            n979 = local write "Phase G"(TRUE ("Phase A")) -> ()
          }
          frame 11 {
            n980 = local read "PhaseA Experiment Option"() -> (w1150:string)
            n981 = local read "PhaseB Experiment Option"() -> (w1137:string)
            n982 = local read "PhaseC Experiment Option"() -> (w1136:string)
            n983 = local read "PhaseD Experiment Option"() -> (w1135:string)
            n984 = local read "PhaseE Experiment Option"() -> (w1134:string)
            n985 = local read "PhaseF Experiment Option"() -> (w1133:string)
            n986 = local write "Phase A Exp Option"(w1150) -> ()
            n987 = local write "Phase B Exp Option"(w1137) -> ()
            n988 = local write "Phase D Exp Option"(w1135) -> ()
            n989 = local write "Phase C Exp Option"(w1136) -> ()
            n990 = local write "Phase E Exp Option"(w1134) -> ()
            n991 = local write "Phase F Exp Option"(w1133) -> ()
            n992 = local write "Phase A"(TRUE ("Phase A")) -> ()
            n993 = local write "Phase C"(TRUE ("Phase A")) -> ()
            n994 = local write "Phase D"(TRUE ("Phase A")) -> ()
            n995 = local write "Phase B"(TRUE ("Phase A")) -> ()
            n996 = local write "Phase E"(TRUE ("Phase A")) -> ()
            n997 = local write "Phase F"(TRUE ("Phase A")) -> ()
            n998 = local read "PhaseG Experiment Option"() -> (w1132:string)
            n999 = local read "PhaseJ Experiment Option"() -> (w1129:string)
            n1000 = local read "PhaseK Experiment Option"() -> (w1128:string)
            n1001 = local write "Phase L Exp Option"("" ("Phase F Exp Option")) -> ()
            n1002 = local read "PhaseH Experiment Option"() -> (w1131:string)
            n1003 = local read "PhaseI Experiment Option"() -> (w1130:string)
            n1004 = local write "Phase K Exp Option"(w1128) -> ()
            n1005 = local write "Phase J Exp Option"(w1129) -> ()
            n1006 = local write "Phase I Exp Option"(w1130) -> ()
            n1007 = local write "Phase G Exp Option"(w1132) -> ()
            n1008 = local write "Phase H Exp Option"(w1131) -> ()
            n1009 = local write "Phase L"(FALSE ("Phase A")) -> ()
            n1010 = local write "Phase K"(TRUE ("Phase A")) -> ()
            n1011 = local write "Phase J"(TRUE ("Phase A")) -> ()
            n1012 = local write "Phase I"(TRUE ("Phase A")) -> ()
            n1013 = local write "Phase H"(TRUE ("Phase A")) -> ()
            n1014 = local write "Phase G"(TRUE ("Phase A")) -> ()
          }
          frame 12 {
            n1015 = local read "PhaseA Experiment Option"() -> (w1175:string)
            n1016 = local read "PhaseB Experiment Option"() -> (w1163:string)
            n1017 = local read "PhaseC Experiment Option"() -> (w1162:string)
            n1018 = local read "PhaseD Experiment Option"() -> (w1161:string)
            n1019 = local read "PhaseE Experiment Option"() -> (w1160:string)
            n1020 = local read "PhaseF Experiment Option"() -> (w1159:string)
            n1021 = local write "Phase A Exp Option"(w1175) -> ()
            n1022 = local write "Phase B Exp Option"(w1163) -> ()
            n1023 = local write "Phase D Exp Option"(w1161) -> ()
            n1024 = local write "Phase C Exp Option"(w1162) -> ()
            n1025 = local write "Phase E Exp Option"(w1160) -> ()
            n1026 = local write "Phase F Exp Option"(w1159) -> ()
            n1027 = local write "Phase A"(TRUE ("Phase A")) -> ()
            n1028 = local write "Phase C"(TRUE ("Phase A")) -> ()
            n1029 = local write "Phase D"(TRUE ("Phase A")) -> ()
            n1030 = local write "Phase B"(TRUE ("Phase A")) -> ()
            n1031 = local write "Phase E"(TRUE ("Phase A")) -> ()
            n1032 = local write "Phase F"(TRUE ("Phase A")) -> ()
            n1033 = local read "PhaseL Experiment Option"() -> (w1153:string)
            n1034 = local read "PhaseG Experiment Option"() -> (w1158:string)
            n1035 = local read "PhaseJ Experiment Option"() -> (w1155:string)
            n1036 = local read "PhaseK Experiment Option"() -> (w1154:string)
            n1037 = local write "Phase L Exp Option"(w1153) -> ()
            n1038 = local read "PhaseH Experiment Option"() -> (w1157:string)
            n1039 = local read "PhaseI Experiment Option"() -> (w1156:string)
            n1040 = local write "Phase K Exp Option"(w1154) -> ()
            n1041 = local write "Phase J Exp Option"(w1155) -> ()
            n1042 = local write "Phase I Exp Option"(w1156) -> ()
            n1043 = local write "Phase G Exp Option"(w1158) -> ()
            n1044 = local write "Phase H Exp Option"(w1157) -> ()
            n1045 = local write "Phase L"(TRUE ("Phase A")) -> ()
            n1046 = local write "Phase K"(TRUE ("Phase A")) -> ()
            n1047 = local write "Phase J"(TRUE ("Phase A")) -> ()
            n1048 = local write "Phase I"(TRUE ("Phase A")) -> ()
            n1049 = local write "Phase H"(TRUE ("Phase A")) -> ()
            n1050 = local write "Phase G"(TRUE ("Phase A")) -> ()
          }
        }
        n1051 = local read "How Many Experimental Phases?"() -> (w823:i32)
        n1052 = local read "Waveform Simulation Jump Filter (Hz)"() -> (w822:dbl)
        n1053 = local read "Waveform Simulation sampling rate (Hz)"() -> (w821:i32)
        n1054 = property class="Clust (strict)"(reference=w854, error in=w839) -> (error out=w851:errorcluster, "Value"=w853:T45)  [unwired: 1 out]
        n1055 = Unbundle By Name(w869) -> ("experiment day folder"=w871:path, "trial name"=w829:string)
        n1056 = Build Path(base path=w871, name or relative path=w829) -> (appended path=w852:path)
        n1057 = Build Path(base path=w852, name or relative path="config.ini") -> (appended path=w849:path)
        n1058 = call "switchSolenoid_topLvl.vi"("which manipulator"=T13."manipulator 1", "error in (no error)"=w851, "solenoidSwitch (T:atm; F: Reg)"=FALSE, "Pressure box control in"=w853) -> ("error out"=w856:errorcluster)  [unwired: 6 in, 1 out]
        n1059 = call "set_status_string.vi"("error in"=w856, "new line?"=TRUE, "status string in"="~~~AUTO RUN ON~~~", "controls array"=w845) -> ("error out"=w868:errorcluster, "controls array out"=w867:refnum<vi>[])  [unwired: 6 in]
        n1060 = Current VI's Path() -> (path=w843:path)
        n1061 = local read "Don't Lift?"() -> (w837:bool)
        n1062 = case shown="False" w837 {
          tunnel: [w929 w930] -> w882
          tunnel: 0.0 ("set holding (mV)") -> [w928 _]
          tunnel: w880 -> [w927 _]
          tunnel: w879 -> [w926 _]
          tunnel: w868 -> [w925 w930]
          frame False {
            n1063 = call "mclamp_set_Vholding_01.vi"("error in (no error)"=w925, "set holding (mV)"=w928, "Error in"=w926, "Multiclamp Handle Out"=w927) -> ("error out"=w929:errorcluster)  [unwired: 6 in, 1 out]
          }
          frame True {
          }
        }
        n1064 = call "Time Delay"("error in (no error)"=w882, "Delay Time (s)"=1.0) -> ("error out"=w878:errorcluster)  [unwired: 9 in]
        n1065 = Select(t="initialCheck" ("ExpPhase"), s=w837, f="preLift" ("ExpPhase")) -> (s? t:f=w866:string)
        n1066 = local read "Lift Cell (T, F-Pull Patch)?"() -> (w883:bool)
        n1067 = call "run_repeatingMembraneTest_pharmabot.vi"("ExpPhase"=w866, "error in"=w878, "data in"=w869, "misc common.stop memtest"=w885, "controls array in"=w867) -> ("error out"=w827:errorcluster, "data out"=w899:T12, "Cell Good?"=w860:bool, "control array out"=w828:refnum<vi>[])  [unwired: 2 in, 1 out]
        n1068 = call "clearOrCalcAllPhaseWaveforms_v02.vi"("How Many Experimental Phases?"=w823, "Clear Waveform?"=TRUE, "error in"=w827, "Waveform Simulation Jump Filter (Hz)"=w822, "Waveform Simulation sampling rate (Hz)"=w821, "ExperimentOptionsCluster"=w824) -> ("error out"=w826:errorcluster)  [unwired: 5 in]
        n1069 = call "condition_control_array_v02.vi"("error in"=w826, "control array in"=w828) -> ("error out"=w847:errorcluster, "control array out"=w848:refnum<vi>[])  [unwired: 8 in]
        n1070 = call "Read and Write Controls to Automatic Config File.vi"("Action"=RWC_Actions."Write", "error in"=w847, "Control References"=w848, "filepath"=w849) -> ("error out"=w846:errorcluster)  [unwired: 7 in]
        n1071 = call "saveExperimentControlArray_v05.vi"("saveFileName"="experimentHeader.txt", "filepath"=w852, "error in"=w846, "mainVI"=w843, "control array in"=w848) -> ("error out"=w831:errorcluster, "control array out"=w844:refnum<vi>[])  [unwired: 5 in]
        n1072 = call "clearOrCalcAllPhaseWaveforms_v02.vi"("How Many Experimental Phases?"=w823, "Clear Waveform?"=FALSE, "error in"=w831, "Waveform Simulation Jump Filter (Hz)"=w822, "Waveform Simulation sampling rate (Hz)"=w821, "ExperimentOptionsCluster"=w824) -> ("error out"=w830:errorcluster)  [unwired: 5 in]
        n1073 = local write "Cell Looks Good?"(w860) -> ()
        n1074 = case shown="False" w837 {
          tunnel: [w1186 w1187] -> w900
          tunnel: w896 -> [w1184 _]
          tunnel: w833 -> [w1183 _]
          tunnel: w895 -> [w1182 _]
          tunnel: w894 -> [w1181 _]
          tunnel: [w1180 w1189] -> w893
          tunnel: w883 -> [w1179 _]
          tunnel: w830 -> [w1178 w1188]
          tunnel: w844 -> [w1177 w1190]
          frame False {
            n1075 = call "liftCellOrPullPatch-v02.vi"("which manipulator"=w1181, "controls array in"=w1177, "LiftCell?"=w1179, "set pressure (mBar)"=-40.0, "error in"=w1178, "common cluster"=w1183, "individual controls in"=w1182, "images"=w1184) -> ("control array out"=w1180:refnum<vi>[], "error out"=w1186:errorcluster)  [unwired: 6 in]
          }
          frame True {
            n1076 = call "set_status_string.vi"("error in"=w1188, "new line?"=TRUE, "status string in"="Not Moving", "controls array"=w1190) -> ("error out"=w1187:errorcluster, "controls array out"=w1189:refnum<vi>[])  [unwired: 6 in]